vi "CRYO_MASTER_FULL_IP.vi"() -> ()   [LabVIEW 2017]
uses:
  LSI218Data.lvclass
  LSI336Data.lvclass
  USBData.lvclass
  6240AData.lvclass
  DMMsData.lvclass
  <vilib>/DAQmx/miscellaneous.llb/DAQmx Fill In Error Info.vi
  <vilib>/DAQmx/create/channels.llb/DAQmx Create Channel (DO-Digital Output).vi
  <vilib>/DAQmx/create/channels.llb/DAQmx Create Channel (AO-Voltage-Basic).vi
  <vilib>/express/express arith-compare/Formula/XNode/ExpressFormulaBlockNode.xnode
  <vilib>/Analysis/NI_AALBase.lvlib
panel:
  out "Graph 12":T1(graph) caption="XY Graph"
  out "Graph 11":T1(graph) caption="XY Graph"
  out "Graph 10":T1(graph) caption="XY Graph"
  in  "Automatic \nScreenshots?":bool=TRUE
  in  "Frontpanel screenshots":bool
  in  "Screenshots interval":i64=3605
  in  "Record interval":i64=10
  out "Cycle #":u32=4959
  in  "Measurement Interval (s)":dbl=1.0
  in  "Stop Button":bool
  in  "?":T2(tab)=enum."DIAGRAM"
  out "RUN Identifier":string="20201002_111738_PreCooling"
  in  "Base Path (screenshots)":path=path "C:/LabVIEW/DATA/Google/TUCAN Experiments/KEK_cryotests_2019-2020/data/screenshots"
  out "error out (USB6210/6218 AOUT)":errorcluster
  in  "AOUT 1 Label":string="KIKUSUI_I"
  in  "AOUT 0 Label":string="KIKUSUI_V"
  in  "DOUT Labels":string[](array[string])=["D_V1_NO", "D_V2_NC", "D_CV1"]
  in  "AOUT for Current CTRL":tag="Dev1/ao1"
  in  "AOUT For Voltage CTRL":tag="Dev1/ao0"
  out "AO task out":refnum<k21>="20201002_111738_PreCooling_AO"
  in  "Analog Out ON?":bool=TRUE
  in  "InstName (USB6218)":string="USB6218"
  in  "USB6218 Config":T3(array[cluster])=[{"Label"="F_1", "FileFormat"="%5.5f", "Active?"=TRUE, "Physical CH"="Dev1/ai0", " terminal\n type"=10083, "ConversionType"={"Type"=enum."SimpleProp", "ConversionParameters"=[0.0, 5.0, 0.0, 500.0]}, "VoltageLimits"=[0.0, 5.0]}, {"Label"="F_2", "FileFormat"="%5.5f", "Active?"=TRUE, "Physical CH"="Dev1/ai1", " terminal\n type"=10083, "ConversionType"={"Type"=enum."SimpleProp", "ConversionParameters"=[0.0, 5.0, 0.0, 200.0]}, "VoltageLimits"=[0.0, 5.0]}, {"Label"="F_3", "FileFormat"="%5.5f", "Active?"=TRUE, "Physical CH"="Dev1/ai2", " terminal\n type"=10083, "ConversionType"={"Type"=enum."SimpleProp", "ConversionParameters"=[0.0, 5.0, 0.0, 200.0]}, "VoltageLimits"=[0.0, 5.0]}, {"Label"="F_4", "FileFormat"="%5.5f", "Active?"=TRUE, "Physical CH"="Dev1/ai3", " terminal\n type"=10083, "ConversionType"={"Type"=enum."SimpleProp", "ConversionParameters"=[0.0, 5.0, 0.0, 500.0]}, "VoltageLimits"=[0.0, 5.0]}, {"Label"="F_5", "FileFormat"="%5.5f", "Active?"=TRUE, "Physical CH"="Dev1/ai4", " terminal\n type"=10083, "ConversionType"={"Type"=enum."SimpleProp", "ConversionParameters"=[0.0, 5.0, 0.0, 500.0]}, "VoltageLimits"=[0.0, 5.0]}, {"Label"="I_CV", "FileFormat"="%3.5f", "Active?"=TRUE, "Physical CH"="Dev1/ai5", " terminal\n type"=10083, "ConversionType"={"Type"=enum."Raw", "ConversionParameters"=[0.0, 0.0, 0.0, 0.0]}, "VoltageLimits"=[0.0, 10.0]}, {"Label"="CV1_answer", "FileFormat"="%3.5f", "Active?"=TRUE, "Physical CH"="Dev1/ai6", " terminal\n type"=10083, "ConversionType"={"Type"=enum."SimpleProp", "ConversionParameters"=[1.0, 5.0, 0.0, 100.0]}, "VoltageLimits"=[0.0, 5.0]}] {"terminal\n type" items=["Default"=-1, "RSE"=10083, "NRSE"=10078, "Differential"=10106, "Pseudodifferential"=12529]}
  out "error out (USB6218)":errorcluster
  out "error out (USB6210/6218 DOUT)":errorcluster
  out "DOUT task out":refnum<k21>="20201002_111738_DO"
  in  "DOUT Physical CH":tag[](array[tag])=["Dev1/port1/line0", "Dev1/port1/line1", "Dev1/port1/line2"]
  in  "Digital Out ON?":bool=TRUE
  in  "USB6210 Config":T3(array[cluster])=[{"Label"="P_ins", "FileFormat"="%5.5e", "Active?"=TRUE, "Physical CH"="Dev2/ai0", " terminal\n type"=10083, "ConversionType"={"Type"=enum."CC-10_LOG", "ConversionParameters"=[0.5, 9.0, 0.0, 1.0]}, "VoltageLimits"=[0.0, 10.0]}, {"Label"="P_4Kres", "FileFormat"="%5.5e", "Active?"=TRUE, "Physical CH"="Dev2/ai1", " terminal\n type"=10083, "ConversionType"={"Type"=enum."SimpleProp", "ConversionParameters"=[1.0, 5.0, 0.0, 200000.0]}, "VoltageLimits"=[0.0, 5.0]}, {"Label"="P_3HeIN", "FileFormat"="%5.5e", "Active?"=TRUE, "Physical CH"="Dev2/ai2", " terminal\n type"=10083, "ConversionType"={"Type"=enum."SimpleProp", "ConversionParameters"=[1.0, 5.0, 0.0, 200000.0]}, "VoltageLimits"=[0.0, 5.0]}, {"Label"="P_SldRTN", "FileFormat"="%5.5e", "Active?"=TRUE, "Physical CH"="Dev2/ai3", " terminal\n type"=10083, "ConversionType"={"Type"=enum."SimpleProp", "ConversionParameters"=[1.0, 5.0, 0.0, 200000.0]}, "VoltageLimits"=[0.0, 5.0]}, {"Label"="P_3Hepot", "FileFormat"="%5.5e", "Active?"=TRUE, "Physical CH"="Dev2/ai4", " terminal\n type"=10083, "ConversionType"={"Type"=enum."SimpleProp", "ConversionParameters"=[0.0, 10.0, 0.0, 133320.0]}, "VoltageLimits"=[0.0, 10.0]}, {"Label"="P_1Kpot", "FileFormat"="%5.5e", "Active?"=TRUE, "Physical CH"="Dev2/ai5", " terminal\n type"=10083, "ConversionType"={"Type"=enum."SimpleProp", "ConversionParameters"=[0.0, 10.0, 0.0, 133320.0]}, "VoltageLimits"=[0.0, 10.0]}, {"Label"="P_Dewar", "FileFormat"="%5.5e", "Active?"=TRUE, "Physical CH"="Dev2/ai6", " terminal\n type"=10083, "ConversionType"={"Type"=enum."SimpleProp", "ConversionParameters"=[1.0, 5.0, 0.0, 200000.0]}, "VoltageLimits"=[0.0, 5.0]}, {"Label"="DP_HEX4", "FileFormat"="%5.5e", "Active?"=TRUE, "Physical CH"="Dev2/ai7", " terminal\n type"=10083, "ConversionType"={"Type"=enum."SimpleProp", "ConversionParameters"=[1.0, 5.0, 0.0, 1000.0]}, "VoltageLimits"=[0.0, 5.0]}, {"Label"="DP_HEX5", "FileFormat"="%5.5e", "Active?"=TRUE, "Physical CH"="Dev2/ai8", " terminal\n type"=10083, "ConversionType"={"Type"=enum."SimpleProp", "ConversionParameters"=[1.0, 5.0, 0.0, 20000.0]}, "VoltageLimits"=[0.0, 5.0]}, {"Label"="L1", "FileFormat"="%5.5f", "Active?"=TRUE, "Physical CH"="Dev2/ai9", " terminal\n type"=10083, "ConversionType"={"Type"=enum."SimpleProp", "ConversionParameters"=[0.0, 10.0, 0.0, 100.0]}, "VoltageLimits"=[0.0, 10.0]}, {"Label"="L2-1", "FileFormat"="%5.5f", "Active?"=TRUE, "Physical CH"="Dev2/ai10", " terminal\n type"=10083, "ConversionType"={"Type"=enum."SimpleProp", "ConversionParameters"=[0.0, 10.0, 0.0, 100.0]}, "VoltageLimits"=[0.0, 10.0]}, {"Label"="L2-2", "FileFormat"="%5.5f", "Active?"=TRUE, "Physical CH"="Dev2/ai11", " terminal\n type"=10083, "ConversionType"={"Type"=enum."SimpleProp", "ConversionParameters"=[0.0, 10.0, 0.0, 100.0]}, "VoltageLimits"=[0.0, 10.0]}, {"Label"="L3", "FileFormat"="%5.5f", "Active?"=TRUE, "Physical CH"="Dev2/ai12", " terminal\n type"=10083, "ConversionType"={"Type"=enum."SimpleProp", "ConversionParameters"=[0.0, 10.0, 0.0, 100.0]}, "VoltageLimits"=[0.0, 10.0]}, {"Label"="P_HEX7OUT", "FileFormat"="%5.5e", "Active?"=TRUE, "Physical CH"="Dev2/ai13", " terminal\n type"=10083, "ConversionType"={"Type"=enum."SimpleProp", "ConversionParameters"=[1.0, 5.0, 0.0, 200000.0]}, "VoltageLimits"=[0.0, 5.0]}, {"Label"="P_IPHe", "FileFormat"="%5.5e", "Active?"=TRUE, "Physical CH"="Dev2/ai14", " terminal\n type"=10083, "ConversionType"={"Type"=enum."CC-10_LOG", "ConversionParameters"=[0.5, 9.0, 0.0, 1.0]}, "VoltageLimits"=[0.0, 10.0]}] {"terminal\n type" items=["Default"=-1, "RSE"=10083, "NRSE"=10078, "Differential"=10106, "Pseudodifferential"=12529]}
  in  "RUN label":string="PreCooling"
  in  "Base Path":path=path "C:/LabVIEW/DATA/Precooling/ScreenShot"
  in  "InstName (USB6210)":string="USB6210"
  out "error out (USB6210)":errorcluster
  out "File Refn USB AO":refnum<file>
  out "File Refn USB DO":refnum<file>
  out "error out (LSI336)":errorcluster
  in  "InstName (LSI336)":string="LSI336"
  in  "FileFormat (336)":string="%4.4f"
  in  "LSI336Settings(X,Y)":T4(array[cluster])=[{"LSIName"="LSi336X", "Labels"=["T1K3-1", "T1K3-2", "T3He5", "T3He8"], "SensorLocations"=[enum."T1K3-1", enum."T1K3-2", enum."T3He5", enum."T3He8"], "Active?"=TRUE, "VISA res. name"="GPIB0::6::INSTR"}, {"LSIName"="LSi336Y", "Labels"=["T3He6-1", "T3He6-2", "T3He7-1", "T3He7-2"], "SensorLocations"=[enum."T3He6-1", enum."T3He6-2", enum."T3He7-1", enum."T3He7-2"], "Active?"=TRUE, "VISA res. name"="GPIB0::2::INSTR"}]
  in  "FileFormat (218)":string="%4.4f"
  in  "InstName (LSI218)":string="LSI218"
  in  "LSI218Settings(A-F)":T4(array[cluster])=[{"LSIName"="LSI218A", "Labels"=["T3He10", "T3He1-1", "TTH3", "TTH4", "TTH1", "TTH2", "T4He1", "T1K1"], "SensorLocations"=[enum."T3He10", enum."T3He1-1", enum."TTH3", enum."TTH4", enum."TTH1", enum."TTH2", enum."T4He1", enum."T1K1"], "Active?"=TRUE, "VISA res. name"="GPIB0::7::INSTR"}, {"LSIName"="LSI218B", "Labels"=["N.C.", "N.C.", "N.C.", "N.C.", "T3He2-1", "T3He2-2", "T3He3", "T3He1-4"], "SensorLocations"=[enum."N.C.", enum."N.C.", enum."N.C.", enum."N.C.", enum."T3He2-1", enum."T3He2-2", enum."T3He3", enum."T3He1-4"], "Active?"=TRUE, "VISA res. name"="GPIB0::4::INSTR"}, {"LSIName"="LSI218C", "Labels"=["T4He3-1", "T4He3-2", "T4He3-3", "T4He3-4", "T4He2-1", "T4He2-2", "T4He4", "T4He5"], "SensorLocations"=[enum."T4He3-1", enum."T4He3-2", enum."T4He3-3", enum."T4He3-4", enum."T4He2-1", enum."T4He2-2", enum."T4He4", enum."T4He5"], "Active?"=TRUE, "VISA res. name"="GPIB0::3::INSTR"}, {"LSIName"="LSI218D", "Labels"=["T4He6", "T4He9", "T3He1-2", "T3He1-3", "T4He7", "T4He8", "T4He10", "T1K6"], "SensorLocations"=[enum."T4He6", enum."T4He9", enum."T3He1-2", enum."T3He1-3", enum."T4He7", enum."T4He8", enum."T4He10", enum."T1K6"], "Active?"=TRUE, "VISA res. name"="GPIB0::5::INSTR"}, {"LSIName"="LSI218E", "Labels"=["TIP1", "N.C.", "TIP2", "N.C.", "TIP3", "TIP4", "TIP5", "N.C."], "SensorLocations"=[enum."TIP1", enum."N.C.", enum."TIP2", enum."N.C.", enum."TIP3", enum."TIP4", enum."TIP5", enum."N.C."], "Active?"=TRUE, "VISA res. name"="GPIB0::11::INSTR"}, {"LSIName"="LSI218F", "Labels"=["T1K2", "T1K4", "T1K5", "T3He4", "T3He9", "TIP6", "N.C.", "N.C."], "SensorLocations"=[enum."T1K2", enum."T1K4", enum."T1K5", enum."T3He4", enum."T3He9", enum."TIP6", enum."N.C.", enum."N.C."], "Active?"=TRUE, "VISA res. name"="GPIB0::8::INSTR"}]
  out "error out (LSI218)":errorcluster
  out "RUN Identifier 2":string="20201002_111738_PreCooling" caption="RUN Identifier"
  out "Graph 3":T1(graph) caption="XY Graph"
  out "Graph 1":T1(graph) caption="XY Graph"
  in  "FIle suffix 4":string="Graph4_1KPot_oscillation"
  in  "Take Screenshot! 4":bool
  in  "Take Screenshot! 3":bool
  in  "Take Screenshot! 2":bool
  in  "Take Screenshot! 1":bool
  in  "FIle suffix 3":string="Graph3_1KPot_oscillation"
  in  "FIle suffix 2":string="Graph2_1KPot_oscillation"
  in  "FIle suffix 1":string="Graph1_1KPot_oscillation"
  in  "log/linear 2":bool
  in  "Tab Control 2":T5(tab)
  in  "Plot selecter (USB6210)\n    1      2     3     4":bool[][](array[boolean])=[[TRUE, FALSE, FALSE, FALSE], [TRUE, FALSE, FALSE, FALSE], [TRUE, FALSE, FALSE, FALSE], [TRUE, FALSE, FALSE, FALSE], [TRUE, FALSE, FALSE, FALSE], [TRUE, FALSE, FALSE, FALSE], [TRUE, FALSE, FALSE, FALSE], [FALSE, TRUE, FALSE, FALSE], [FALSE, TRUE, FALSE, FALSE], [FALSE, TRUE, FALSE, FALSE], [FALSE, TRUE, FALSE, FALSE], [FALSE, TRUE, FALSE, FALSE], [FALSE, TRUE, FALSE, FALSE], [TRUE, FALSE, FALSE, FALSE], [FALSE, FALSE, FALSE, FALSE], [FALSE, FALSE, FALSE, FALSE]]
  out "All Labels (USB6210)":string[](array[string])=["P_ins", "P_4Kres", "P_3HeIN", "P_SldRTN", "P_3Hepot", "P_1Kpot", "P_Dewar", "DP_HEX4", "DP_HEX5", "L1", "L2-1", "L2-2", "L3", "P_HEX7OUT"]
  out "Last Data \n(USB6210)":dbl[](array[numeric])=[0.00015623126743967978, 102646.15993978488, 3637.6504873774197, 101891.36809168091, 4295.356268996977, 845.3614360135382, 101097.11052150725, -5.334954304017453, 66.29225516513348, 99.98613335417497, 67.02762914376657, 60.52032349741818, 48.99728244152156, 103856.45826569716] format="%#_6e"
  out "Time of Last Measurement (USB6210)":timestamp=timestamp(3684454864.3849993 s since 1904-01-01)
  out "USB6210 Status":T6(ring)=enum."Ready"
  out "Last Vol\n(USB6210)":dbl[](array[numeric])=[5.596883978015126, 3.0529231987956975, 1.0727530097475484, 3.0378273618336182, 0.32218393856863015, 0.06340844854586995, 3.021942210430145, 0.9786601827839302, 1.0132584510330267, 9.998613335417497, 6.702762914376658, 6.052032349741818, 4.899728244152156, 3.077129165313943] format="%_5f"
  out "Time of Last Measurement (USB6218)":timestamp=timestamp(3684454864.391945 s since 1904-01-01)
  out "USB6218 Status":T6(ring)=enum."Ready"
  out "Last Vol \n(USB6218)":dbl[](array[numeric])=[0.4328486013755781, 0.2856827409675284, 0.008941174623972741, -0.06513496143958923, 0.9306675842076008, -6.309670101250775e-05, -0.00046218726464117564] format="%_5f"
  out "Last Data \n(USB6218)":dbl[](array[numeric])=[43.284860137557814, 11.427309638701136, 0.3576469849589097, -6.513496143958923, 93.06675842076008, -6.309670101250775e-05, -25.011554681616026] format="%#_6e"
  out "All Labels (USB6218)":string[](array[string])=["F_1", "F_2", "F_3", "F_4", "F_5", "I_CV", "CV1_answer"]
  in  "Plot selecter (USB6218)\n    1      2     3     4":bool[][](array[boolean])=[[FALSE, FALSE, TRUE, FALSE], [FALSE, FALSE, TRUE, FALSE], [FALSE, FALSE, TRUE, FALSE], [FALSE, FALSE, TRUE, FALSE], [FALSE, FALSE, TRUE, FALSE], [FALSE, FALSE, TRUE, FALSE], [FALSE, FALSE, FALSE, FALSE], [FALSE, FALSE, TRUE, FALSE], [FALSE, FALSE, TRUE, FALSE], [FALSE, FALSE, FALSE, TRUE], [FALSE, FALSE, FALSE, TRUE], [FALSE, FALSE, FALSE, TRUE], [FALSE, FALSE, FALSE, TRUE], [FALSE, FALSE, FALSE, FALSE], [FALSE, FALSE, FALSE, FALSE], [FALSE, FALSE, FALSE, FALSE]]
  out "Time of Last Measurement (LSI218)":timestamp=timestamp(3684454864.3849993 s since 1904-01-01)
  out "LSI218 Status":T7(ring)=enum."Measuring"
  out "Last Data \nLSI218 (1)":dbl[](array[numeric])=[174.86, 119.03, 131.93, 123.27, 24.68, 25.174, 4.416, 4.607, 30.0, 0.0, 0.0, 0.0, 66.96, 49.172, 4.786, 225.14, 190.27, 196.43, 244.83, 249.59, 17.993, 18.993, 22.964, 24.809]
  out "Labels LSI218 (1)":string[](array[string])=["T3He10", "T3He1-1", "TTH3", "TTH4", "TTH1", "TTH2", "T4He1", "T1K1", "N.C.", "N.C.", "N.C.", "N.C.", "T3He2-1", "T3He2-2", "T3He3", "T3He1-4", "T4He3-1", "T4He3-2", "T4He3-3", "T4He3-4", "T4He2-1", "T4He2-2", "T4He4", "T4He5"]
  in  "Plot selecter LSI218(1)\n    1      2     3     4":bool[][](array[boolean])=[[FALSE, FALSE, FALSE, FALSE], [FALSE, FALSE, FALSE, FALSE], [FALSE, FALSE, FALSE, TRUE], [FALSE, FALSE, FALSE, TRUE], [FALSE, FALSE, FALSE, TRUE], [FALSE, FALSE, FALSE, TRUE], [FALSE, FALSE, FALSE, TRUE], [FALSE, FALSE, FALSE, TRUE], [FALSE, FALSE, FALSE, FALSE], [FALSE, FALSE, FALSE, FALSE], [FALSE, FALSE, FALSE, FALSE], [FALSE, FALSE, FALSE, FALSE], [FALSE, FALSE, FALSE, TRUE], [FALSE, FALSE, FALSE, TRUE], [FALSE, FALSE, FALSE, FALSE], [FALSE, FALSE, FALSE, FALSE], [FALSE, FALSE, FALSE, TRUE], [FALSE, FALSE, FALSE, TRUE], [FALSE, FALSE, FALSE, TRUE], [FALSE, FALSE, FALSE, TRUE], [FALSE, FALSE, FALSE, TRUE], [FALSE, FALSE, FALSE, TRUE], [FALSE, FALSE, FALSE, TRUE], [FALSE, FALSE, FALSE, FALSE]]
  out "Active?\n (1)":bool[](array[boolean])=[TRUE, TRUE, TRUE, TRUE, TRUE, TRUE, TRUE, TRUE, TRUE, TRUE, TRUE, TRUE, TRUE, TRUE, TRUE, TRUE, TRUE, TRUE, TRUE, TRUE, TRUE, TRUE, TRUE, TRUE]
  out "Labels LSI218 (2)":string[](array[string])=["T4He6", "T4He9", "T3He1-2", "T3He1-3", "T4He7", "T4He8", "T4He10", "T1K6", "TIP1", "N.C.", "TIP2", "N.C.", "TIP3", "TIP4", "TIP5", "N.C.", "T1K2", "T1K4", "T1K5", "T3He4", "T3He9", "TIP6", "N.C.", "N.C."]
  out "Active?\n(2)":bool[](array[boolean])=[TRUE, TRUE, TRUE, TRUE, TRUE, TRUE, TRUE, TRUE, TRUE, TRUE, TRUE, TRUE, TRUE, TRUE, TRUE, TRUE, TRUE, TRUE, TRUE, TRUE, TRUE, TRUE, TRUE, TRUE]
  out "Last Data \nLSI218 (2)":dbl[](array[numeric])=[26.249, 111.49, 133.91, 219.75, 133.21, 138.02, 218.7, 58.064, 250.36, 0.0, 110.28, 688.49, 56.993, 6.89, 10.053, 688.58, 1.955, 1.89, 4.175, 2.013, 2.158, 18.589, 0.433, 0.0]
  in  "Plot selecter LSI218(2)\n    1      2     3     4":bool[][](array[boolean])=[[FALSE, FALSE, FALSE, FALSE], [FALSE, FALSE, FALSE, FALSE], [FALSE, FALSE, FALSE, FALSE], [FALSE, FALSE, FALSE, FALSE], [FALSE, FALSE, FALSE, FALSE], [FALSE, FALSE, FALSE, FALSE], [FALSE, FALSE, FALSE, FALSE], [FALSE, FALSE, FALSE, FALSE], [FALSE, FALSE, FALSE, FALSE], [FALSE, FALSE, FALSE, FALSE], [FALSE, FALSE, FALSE, FALSE], [FALSE, FALSE, FALSE, FALSE], [FALSE, FALSE, FALSE, FALSE], [FALSE, FALSE, FALSE, FALSE], [FALSE, FALSE, FALSE, FALSE], [FALSE, FALSE, FALSE, FALSE], [FALSE, FALSE, FALSE, TRUE], [FALSE, FALSE, FALSE, TRUE], [FALSE, FALSE, FALSE, TRUE], [FALSE, FALSE, FALSE, FALSE], [FALSE, FALSE, FALSE, FALSE], [FALSE, FALSE, FALSE, FALSE], [FALSE, FALSE, FALSE, FALSE], [FALSE, FALSE, FALSE, FALSE]]
  in  "Plot selecter LSI336 \n     1      2     3     4":bool[][](array[boolean])=[[FALSE, FALSE, FALSE, TRUE], [FALSE, FALSE, FALSE, TRUE], [FALSE, FALSE, FALSE, TRUE], [FALSE, FALSE, FALSE, TRUE], [FALSE, FALSE, FALSE, TRUE], [FALSE, FALSE, FALSE, TRUE], [FALSE, FALSE, FALSE, TRUE], [FALSE, FALSE, FALSE, TRUE]]
  out "Time of Last Measurement (LSI336)":timestamp=timestamp(3684454864.3849993 s since 1904-01-01)
  out "Last Data \nLSI336":dbl[](array[numeric])=[1.5337, 1.5296, 1.8153, 2.1079, 2.1163, 2.122, 2.1204, 2.1198]
  out "Active?\n(LSI336)":bool[](array[boolean])=[TRUE, TRUE, TRUE, TRUE, TRUE, TRUE, TRUE, TRUE]
  out "Labels LSI336":string[](array[string])=["T1K3-1", "T1K3-2", "T3He5", "T3He8", "T3He6-1", "T3He6-2", "T3He7-1", "T3He7-2"]
  out "LSI336 Status":T7(ring)=enum."Measuring"
  in  "log/linear 1":bool=TRUE
  out "Graph 2":T1(graph) caption="XY Graph"
  out "Graph 4":T1(graph) caption="XY Graph"
  in  "log/linear 4":bool
  in  "log/linear 3":bool
  out "RUN Identifier 3":string="20201002_111738_PreCooling" caption="RUN Identifier"
  out "RUN Identifier 4":string="20201002_111738_PreCooling" caption="RUN Identifier"
  out "Fill (false)":bool=TRUE
  in  "Fill state":bool
  out "state 1 (false)":bool=TRUE
  out "state 1":bool
  out "state 2":bool
  out "state 2 (false)":bool=TRUE
  out "Status V2 CTRL":enum16{"Pressurize", "Release"}(ring)
  out "Status V1 CTRL":enum16{"Pressurize", "Release"}(ring)
  out "Lav (%)":dbl=71.20324134668614 format="%0.2f"
  out "Lstd":dbl=0.006921328322954857 format="%0.2f"
  out "Last N M.A. Levels":dbl[](array[numeric])=[71.21069849829522, 71.21168495646573, 71.21563078793135, 71.20971204069737, 71.19803895584928, 71.19672367846871, 71.19162697956635, 71.19771013641974, 71.20247801612076, 71.19951864246737, 71.19738131717675, 71.2023136066108, 71.20675266705979, 71.20510857047677] format="%_5e"
  out "Lstd history":dbl(graph)=0.007035562623226079
  out "Lav history":dbl(graph)=71.20346447405132
  out "Target Index (L)":i32=12
  in  "Auto Fll\nHe level label":string="L3"
  out "Target Index (P)":i32=6
  in  "Auto Fll\nDewar P. label":string="P_Dewar"
  out "He Level":T8(graph)=[{"TimeArray"=[timestamp(3684373440.273899 s since 1904-01-01), timestamp(3684373441.2730346 s since 1904-01-01), timestamp(3684373442.273437 s since 1904-01-01), timestamp(3684373443.273284 s since 1904-01-01), timestamp(3684373444.272991 s since 1904-01-01), timestamp(3684373445.2752414 s since 1904-01-01), timestamp(3684373446.273977 s since 1904-01-01), timestamp(3684373447.275109 s since 1904-01-01), timestamp(3684373448.275254 s since 1904-01-01), timestamp(3684373449.2756577 s since 1904-01-01), timestamp(3684373450.4052033 s since 1904-01-01), timestamp(3684373451.404408 s since 1904-01-01), timestamp(3684373452.4054728 s since 1904-01-01), timestamp(3684373453.4055552 s since 1904-01-01)], "Filtered X"=[71.22204276382959, 71.21217818635228, 71.21283582343595, 71.19179138917168, 71.17535042443726, 71.20691707682998, 71.19244902782646, 71.21612401658533, 71.1944219432413, 71.1950795822164, 71.18389972666398, 71.2358531743215, 71.21217818503723, 71.18850319588435]}, {"TimeArray"=[timestamp(3684373440.273899 s since 1904-01-01), timestamp(3684373441.2730346 s since 1904-01-01), timestamp(3684373442.273437 s since 1904-01-01), timestamp(3684373443.273284 s since 1904-01-01), timestamp(3684373444.272991 s since 1904-01-01), timestamp(3684373445.2752414 s since 1904-01-01), timestamp(3684373446.273977 s since 1904-01-01), timestamp(3684373447.275109 s since 1904-01-01), timestamp(3684373448.275254 s since 1904-01-01), timestamp(3684373449.2756577 s since 1904-01-01), timestamp(3684373450.4052033 s since 1904-01-01), timestamp(3684373451.404408 s since 1904-01-01), timestamp(3684373452.4054728 s since 1904-01-01), timestamp(3684373453.4055552 s since 1904-01-01)], "Filtered X"=[71.21069849829522, 71.21168495646573, 71.21563078793135, 71.20971204069737, 71.19803895584928, 71.19672367846871, 71.19162697956635, 71.19771013641974, 71.20247801612076, 71.19951864246737, 71.19738131717675, 71.2023136066108, 71.20675266705979, 71.20510857047677]}] caption="XY Graph"
  in  "P_safelimit_high (Pa)":dbl=300000.0 format="%_4e"
  in  "P_safelimit_low (Pa)":dbl=100.0 format="%_4e"
  in  "Auto Fill ON?":bool
  out "Pstd history":dbl(graph)=271.0714505072834
  out "Pav history":dbl(graph)=125228.66056725154
  in  "Mov. Avg Interval":i64=4
  in  "V2 (N.C.)":bool
  in  "V1 (N.O.)":bool=TRUE
  in  "N for sampling":i64=7
  in  "L_low (%)":dbl=60.0 format="%_3f"
  in  "L_high (%)":dbl=80.0 format="%_3g"
  in  "P_2_low (Pa)":dbl=125000.0 format="%_4e"
  in  "P_1_low (Pa)":dbl=135000.0 format="%_4g"
  in  "P_2_high (Pa)":dbl=135000.0 format="%_4e"
  in  "P_1_high (Pa)":dbl=140000.0 format="%_4e"
  out "Dewar Pressure":T8(graph)=[{"TimeArray"=[timestamp(3684373440.273899 s since 1904-01-01), timestamp(3684373441.2730346 s since 1904-01-01), timestamp(3684373442.273437 s since 1904-01-01), timestamp(3684373443.273284 s since 1904-01-01), timestamp(3684373444.272991 s since 1904-01-01), timestamp(3684373445.2752414 s since 1904-01-01), timestamp(3684373446.273977 s since 1904-01-01), timestamp(3684373447.275109 s since 1904-01-01), timestamp(3684373448.275254 s since 1904-01-01), timestamp(3684373449.2756577 s since 1904-01-01), timestamp(3684373450.4052033 s since 1904-01-01), timestamp(3684373451.404408 s since 1904-01-01), timestamp(3684373452.4054728 s since 1904-01-01), timestamp(3684373453.4055552 s since 1904-01-01)], "Filtered X"=[126288.14675345753, 125406.72915551426, 125684.63887820412, 125234.06378922188, 125026.86502899571, 125252.15243360576, 124413.49040192305, 124206.29196931639, 125817.83836590881, 125184.73094394046, 125132.10848420773, 125707.66108196737, 125227.48582278784, 126493.70118827428]}, {"TimeArray"=[timestamp(3684373440.273899 s since 1904-01-01), timestamp(3684373441.2730346 s since 1904-01-01), timestamp(3684373442.273437 s since 1904-01-01), timestamp(3684373443.273284 s since 1904-01-01), timestamp(3684373444.272991 s since 1904-01-01), timestamp(3684373445.2752414 s since 1904-01-01), timestamp(3684373446.273977 s since 1904-01-01), timestamp(3684373447.275109 s since 1904-01-01), timestamp(3684373448.275254 s since 1904-01-01), timestamp(3684373449.2756577 s since 1904-01-01), timestamp(3684373450.4052033 s since 1904-01-01), timestamp(3684373451.404408 s since 1904-01-01), timestamp(3684373452.4054728 s since 1904-01-01), timestamp(3684373453.4055552 s since 1904-01-01)], "Filtered X"=[125428.10696888957, 125511.97316498918, 125422.7625555792, 125653.39464409945, 125338.074212984, 125299.43003250686, 124981.6429134366, 124724.69995846022, 124922.4432926885, 124905.58792027218, 125085.24244084334, 125460.58471900609, 125312.99658322585, 125640.23914430931]}] caption="XY Graph"
  out "Last N M.A. Pressures":dbl[](array[numeric])=[125428.10696888957, 125511.97316498918, 125422.7625555792, 125653.39464409945, 125338.074212984, 125299.43003250686, 124981.6429134366, 124724.69995846022, 124922.4432926885, 124905.58792027218, 125085.24244084334, 125460.58471900609, 125312.99658322585, 125640.23914430931] format="%_5e"
  out "Pav (Pa)":dbl=125263.36989652073 format="%0.4e"
  out "Pstd":dbl=291.18311466125465 format="%0.4e"
  out "File Refn DewarCTRL":refnum<file>
  out "Error Out (Dewar CTRL":errorcluster
  in  "update values":bool
  out "Monitor Current (mA)":dbl=-0.5520142344653531 min=0.0 max=1.9 format="%_4e"
  in  "update current":bool
  out "USB AOUT":dbl[](array[numeric])=[12.0, 4.0, 0.18461538461538463, 0.06969546425555169]
  out "Graph 7":T9(graph) caption="XY Graph"
  in  "upper limit (V)\n (Kikusui)":dbl=12.0 format="%_3f"
  in  "lower limit (V) \n(Kikusui)":dbl format="%_3f"
  in  "lower limit (mA) \n(Kikusui)":dbl=4.0 format="%_3f"
  in  "upper limit (mA)\n (Kikusui)":dbl=40.0 format="%_3f"
  in  "lower limit (mA)":dbl=4.0 format="%_3f"
  in  "SetCurrent 2 (mA)":dbl=4.0 min=4.0 max=500.0 format="%_3f"
  in  "upper limit (mA)":dbl=500.0 format="%_3f"
  out "error out (KIKUSI CTRL)":errorcluster
  out "ActualVoltage (V)":dbl[](array[numeric]) format="%_6g"
  out "ActualCurrent (A)":dbl[](array[numeric])=[0.01, 0.0] format="%_3e"
  in  "SetCurrent 1 (mA)":dbl=4.0 min=4.0 max=500.0 format="%_3g"
  in  "Output\n (ADCMT)":bool[](array[boolean])=[FALSE, FALSE]
  out "error out (ADCMT6420A)":errorcluster
  in  "Voltage limits (V)":dbl[](array[numeric])=[12.0, 12.0] format="%_3f"
  in  "CtrlLabels":string[](array[string])=["CV2", "CV3"]
  in  "VISA":refnum<visa-resource-name>[](array[refnum])=["GPIB0::1::INSTR", "GPIB0::12::INSTR"]
  out "Initialized?":bool
  in  "InstName":string="ADCMT6240"
  out "Graph 6":T8(graph)=[{"TimeArray"=[timestamp(3684448950.65012 s since 1904-01-01), timestamp(3684448954.168732 s since 1904-01-01), timestamp(3684448960.15376 s since 1904-01-01)], "Filtered X"=[0.8, 0.8, 0.01]}, {"TimeArray"=[timestamp(3684448950.65012 s since 1904-01-01), timestamp(3684448954.168732 s since 1904-01-01), timestamp(3684448960.15376 s since 1904-01-01)], "Filtered X"=[0.0, 0.0, 0.0]}, {"TimeArray"=[timestamp(3684448950.65012 s since 1904-01-01), timestamp(3684448954.168732 s since 1904-01-01), timestamp(3684448960.15376 s since 1904-01-01)], "Filtered X"=[0.8, 0.8, 0.01]}, {"TimeArray"=[timestamp(3684448950.65012 s since 1904-01-01), timestamp(3684448954.168732 s since 1904-01-01), timestamp(3684448960.15376 s since 1904-01-01)], "Filtered X"=[0.0, 0.0, 0.0]}] caption="XY Graph"
  in  "Initialize":bool
  in  "CONTROL KIKUSUI?":bool=TRUE
  in  "OUTPUT\n(Kikusui)":bool
  in  "Set Voltage (V)\n (Kikusui)":dbl=12.0 min=0.0 max=12.0 format="%_3g"
  in  "Set Current (mA)\n (Kikusui)":dbl=4.0 min=4.0 max=40.0 format="%_3g"
  out "RUN Identifier 5":string="20201002_111738_PreCooling" caption="RUN Identifier"
  in  "Measure DMMs?":bool
  out "DMMsLabels":string[](array[string])=["V_H2", "V_H4", "I_H2", "I_H4"]
  out "Active?":bool[](array[boolean])=[TRUE, FALSE, TRUE, FALSE]
  out "DMM LastMeasurements":dbl[](array[numeric])=[2.6334599999999997e-05, 0.0, 0.0, 0.0]
  out "Graph DMMs 2":T1(graph) caption="XY Graph"
  out "DMMFileName":string="20201001_162428_PreCooling_DMMs_20201001_162516.csv"
  out "error out (DMMs)":errorcluster
  out "cycle # (DMMs)":i32=10009
  in  "DMMsConfig":T10(array[cluster])=[{"Label"="V_H2", "Active?"=TRUE, "VISA resource name"="GPIB0::22::INSTR", "Device"=enum."Agilent34401A", "Measurement"=enum."DC Volts", "FileFormat"="%4.6e"}, {"Label"="V_H4", "Active?"=FALSE, "VISA resource name"="USB0::0x1334::0x0204::262800451::INSTR", "Device"=enum."ADCMT7351", "Measurement"=enum."DC Volts", "FileFormat"="%4.6e"}, {"Label"="I_H2", "Active?"=TRUE, "VISA resource name"="USB0::0x1334::0x0204::262800066::INSTR", "Device"=enum."ADCMT7351", "Measurement"=enum."DC Currents", "FileFormat"="%4.4e"}, {"Label"="I_H4", "Active?"=FALSE, "VISA resource name"="GPIB0::23::INSTR", "Device"=enum."HP3478A", "Measurement"=enum."DC Currents", "FileFormat"="%4.4e"}]
  in  "Measurement Interval DMMs (ms)":i64=500
  in  "InstName DMMs":string="DMMs"
  in  "Initialize (DMMs)":bool
  out "Graph DMMs 1":T1(graph) caption="XY Graph"
  out "error out (DMM graphs)":errorcluster
  in  "Sample #":i32=5
  in  "IPHe pressure":string="P_IPHe"
  out "P (IPHe)":dbl=102813.89149070326 format="%_4e"
  out "P_IPHe":dbl=102813.89149070326 format="%_4e"
  out "P_HEX7OUT":dbl=102813.89149070326 format="%_4e"
  out "P (HEX7 out)":dbl=102813.89149070326 format="%_4e"
  out "DP HEX5":dbl=83.0651823977413 format="%_4e"
  out "DP_HEX5":dbl=83.0651823977413 format="%_4e"
  in  "Diff pressure HEX5":string="DP_HEX5"
  out "3He pot level":dbl=100.01835834612064 format="%_4f"
  in  "3He pot":string="L1"
  out "He level (3He)":dbl(slide)=100.01835834612064 scale=0.0..100.0
  out "He level (1K) b":dbl(slide)=60.44995659847142 scale=0.0..100.0
  out "He level (1K)":dbl(slide)=66.98422510636897 scale=0.0..100.0
  out "He level (4K)":dbl(slide)=48.990048499529806 scale=0.0..100.0
  out "1K pot(b1)":dbl=60.44995659847142 format="%_4f"
  in  "1K pot (b)":string="L2-2"
  in  "1K pot level":string="L2-1"
  out "L(1K) (a1)":dbl=66.98422510636897 format="%_4f"
  in  "SensorLocation 2":T11(ring)=enum."T3He5"
  out "Temperature 2":dbl=1.7995
  out "DP HEX4":dbl=-5.3760643808830615 format="%_4e"
  in  "Diff pressure HEX4":string="DP_HEX4"
  out "V2":bool
  out "V1":bool=TRUE
  out "F5 (3He pump ex.)":dbl=93.69145685771404 format="%_4f"
  out "F4 (3He in to HEX7)":dbl=-6.1879951345084425 format="%_3f"
  out "F3 (4He rtn flw via HEX7)":dbl=0.443132092574638 format="%_4f"
  out "F1 (1K pump exhaust) flow":dbl=43.19279928269202 format="%_4f"
  out "P (Dewar)":dbl=101207.2871705193 format="%_4e"
  out "P (1K pot)":dbl=854.1288946139209 format="%_4e"
  out "P (3He pot)":dbl=4268.177149245784 format="%_4e"
  out "P (shield return)":dbl=102073.89943522238 format="%_4e"
  out "P (3He IN)":dbl=3879.377992445654 format="%_4e"
  out "P (4K reservoir)":dbl=102544.20548859666 format="%_4e"
  out "P (insulation)":dbl=0.00015646802075869302 format="%_4e"
  in  "3He pump exhaust flow":string="F_5"
  out "F_5":dbl=93.69145685771404 format="%_4f"
  in  "3He incoming flow into HEX7":string="F_4"
  out "F_4":dbl=-6.1879951345084425 format="%_4f"
  out "F_3":dbl=0.443132092574638 format="%_4f"
  in  "4He return flow from HEX7":string="F_3"
  out "F_2":dbl=11.32341237657438 format="%_4f"
  in  "Shield flow":string="F_2"
  out "P_SldRTN":dbl=102073.89943522238 format="%_4e"
  in  "3He pot pressure":string="P_3Hepot"
  out "P_3Hepot":dbl=4268.177149245784 format="%_4e"
  in  "Shield return press.":string="P_SldRTN"
  out "F_1":dbl=43.19279928269202 format="%_4f"
  in  "1K pump exhaust flow":string="F_1"
  out "P_Dewar":dbl=101207.2871705193 format="%_4e"
  in  "Dewar pressure":string="P_Dewar"
  out "P_1Kpot":dbl=854.1288946139209 format="%_4e"
  in  "1Kpot pressure":string="P_1Kpot"
  out "P_3HeIN":dbl=3879.377992445654 format="%_4e"
  in  "3He inlet pressure":string="P_3HeIN"
  in  "4K reservoir pressure":string="P_4Kres"
  out "P_4Kres":dbl=102544.20548859666 format="%_4e"
  out "P_ins":dbl=0.00015646802075869302 format="%_4e"
  in  "Insulation vacuum":string="P_ins"
  out "T3He7-1/6-2 (3He pot) 2":dbl=2.1199 format="%_4f"
  out "T3He7-1/7-2 (HEX1)":dbl=2.1206 format="%_4f"
  out "T3He6-1/6-2 (3He pot) 2":dbl=2.1224 format="%_4f"
  out "T3He6-1/6-2 (HEX1)":dbl=2.1167 format="%_4f"
  out "T1K3-1/3-2 (1K pot) 2":dbl=1.53 format="%_4f"
  out "T1K3-1/3-2 (1K pot)":dbl=1.5341 format="%_4f"
  out "T4He1 (4K reservoir )":dbl=4.418 format="%_4f"
  out "Temperature 1":dbl=25.175
  in  "SensorLocation 1":T11(ring)=enum."TTH2"
  out "TIP7":dbl format="%_4g"
  out "T3He6-2":dbl=2.1224 format="%_4g"
  out "T3He7-2":dbl=2.1199 format="%_4g"
  out "T3He6-1":dbl=2.1167 format="%_4g"
  out "T3He4":dbl=2.021 format="%_4g"
  out "T3He7-1":dbl=2.1206 format="%_4g"
  out "T3He8":dbl=2.1078 format="%_4g"
  out "T3He5":dbl=1.7995 format="%_4g"
  out "T1K3-2":dbl=1.53 format="%_4g"
  out "T1K3-1":dbl=1.5341 format="%_4g"
  out "TIP6":dbl=18.591 format="%_4g"
  out "T3He9":dbl=2.146 format="%_4g"
  out "T1K5":dbl=4.181 format="%_4g"
  out "T1K4":dbl=1.897 format="%_4g"
  out "T1K2":dbl=1.952 format="%_4g"
  out "TIP5":dbl=10.064 format="%_4g"
  out "TIP4":dbl=6.894 format="%_4g"
  out "TIP3":dbl=56.992 format="%_4g"
  out "TIP2":dbl=110.28 format="%_4g"
  out "TIP1":dbl=250.37 format="%_4g"
  out "T1K6":dbl=58.037 format="%_4g"
  out "T4He10":dbl=218.68 format="%_4g"
  out "T4He8":dbl=138.02 format="%_4g"
  out "T4He7":dbl=133.22 format="%_4g"
  out "T3He1-3":dbl=219.72 format="%_4g"
  out "T3He1-2":dbl=133.83 format="%_4g"
  out "T4He9":dbl=111.48 format="%_4g"
  out "T4He6":dbl=26.241 format="%_4g"
  out "T4He5":dbl=24.814 format="%_4g"
  out "T4He4":dbl=22.962 format="%_4g"
  out "T4He2-2":dbl=19.013 format="%_4g"
  out "T4He2-1":dbl=17.972 format="%_4g"
  out "T4He3-4":dbl=249.58 format="%_4g"
  out "T4He3-3":dbl=244.82 format="%_4g"
  out "T4He3-2":dbl=196.4 format="%_4g"
  out "T4He3-1":dbl=190.21 format="%_4g"
  out "T3He1-4":dbl=225.11 format="%_4g"
  out "T3He3":dbl=4.771 format="%_4g"
  out "T3He2-2":dbl=49.183 format="%_4g"
  out "T3He2-1":dbl=66.962 format="%_4g"
  out "T1K1":dbl=4.591 format="%_4g"
  out "T4He1":dbl=4.418 format="%_4g"
  out "TTH1":dbl=24.68 format="%_4g"
  out "TTH2":dbl=25.175 format="%_4g"
  out "TTH4":dbl=123.27 format="%_4g"
  out "TTH3":dbl=131.91 format="%_4g"
  out "T3He1-1":dbl=118.93 format="%_4g"
  out "T3He10":dbl=174.85 format="%_4g"
  out "F2 (shield flow)":dbl=11.32341237657438 format="%_4f"
  out "DP_HEX4":dbl=-5.3760643808830615 format="%_4e"
  in  "4K reservoir level":string="L3"
  out "L3":dbl=48.990048499529806 format="%_4f"
  out "RUN Identifier 6":string="20201002_111738_PreCooling" caption="RUN Identifier"
  in  "HEX7 out pressure":string="P_HEX7OUT"
  out "Series 1":string[](array[string])=["P_ins", "P_4Kres", "P_3HeIN", "P_SldRTN", "P_3Hepot", "P_1Kpot", "P_Dewar", "P_HEX7OUT"]
  out "Series 2":string[](array[string])=["DP_HEX4", "DP_HEX5", "L1", "L2-1", "L2-2", "L3"]
  out "Series 3":string[](array[string])=["F_1", "F_2", "F_3", "F_4", "F_5", "I_CV"]
  out "Series 4":string[](array[string])=["TTH3", "TTH4", "TTH1", "TTH2", "T4He1", "T1K1", "T3He2-1", "T3He2-2", "T4He3-1", "T4He3-2", "T4He3-3", "T4He3-4", "T4He2-1", "T4He2-2", "T4He4", "T1K2", "T1K4", "T1K5", "T1K3-1", "T1K3-2", "T3He5", "T3He8", "T3He6-1", "T3He6-2", "T3He7-1", "T3He7-2"]
  out "Plot errors":errorcluster
  out "LastMeasurementConfig (218)":T12(array[cluster])=[{"LSIName"="LSI218A", "Active?"=TRUE, "LastData"=[174.86, 119.03, 131.93, 123.27, 24.68, 25.174, 4.416, 4.607], "Labels"=["T3He10", "T3He1-1", "TTH3", "TTH4", "TTH1", "TTH2", "T4He1", "T1K1"]}, {"LSIName"="LSI218B", "Active?"=TRUE, "LastData"=[30.0, 0.0, 0.0, 0.0, 66.96, 49.172, 4.786, 225.14], "Labels"=["N.C.", "N.C.", "N.C.", "N.C.", "T3He2-1", "T3He2-2", "T3He3", "T3He1-4"]}, {"LSIName"="LSI218C", "Active?"=TRUE, "LastData"=[190.27, 196.43, 244.83, 249.59, 17.993, 18.993, 22.964, 24.809], "Labels"=["T4He3-1", "T4He3-2", "T4He3-3", "T4He3-4", "T4He2-1", "T4He2-2", "T4He4", "T4He5"]}, {"LSIName"="LSI218D", "Active?"=TRUE, "LastData"=[26.249, 111.49, 133.91, 219.75, 133.21, 138.02, 218.7, 58.064], "Labels"=["T4He6", "T4He9", "T3He1-2", "T3He1-3", "T4He7", "T4He8", "T4He10", "T1K6"]}, {"LSIName"="LSI218E", "Active?"=TRUE, "LastData"=[250.36, 0.0, 110.28, 688.49, 56.993, 6.89, 10.053, 688.58], "Labels"=["TIP1", "N.C.", "TIP2", "N.C.", "TIP3", "TIP4", "TIP5", "N.C."]}, {"LSIName"="LSI218F", "Active?"=TRUE, "LastData"=[1.955, 1.89, 4.175, 2.013, 2.158, 18.589, 0.433, 0.0], "Labels"=["T1K2", "T1K4", "T1K5", "T3He4", "T3He9", "TIP6", "N.C.", "N.C."]}]
  out "DataArrayConv (USB6210)":dbl[][](array[numeric])
  out "LastMeasurementConfig (336)":T12(array[cluster])=[{"LSIName"="LSi336X", "Active?"=TRUE, "LastData"=[1.5337, 1.5296, 1.8153, 2.1079], "Labels"=["T1K3-1", "T1K3-2", "T3He5", "T3He8"]}, {"LSIName"="LSi336Y", "Active?"=TRUE, "LastData"=[2.1163, 2.122, 2.1204, 2.1198], "Labels"=["T3He6-1", "T3He6-2", "T3He7-1", "T3He7-2"]}]
  out "DataArrayConv (USB6218)":dbl[][](array[numeric])
  out "TimeArray (USB6218)":timestamp[](array[timestamp])
  out "Data Array sizes (6210)":i32[](array[numeric])=[4959, 14]
  out "DataArraySize (6218)":i32[](array[numeric])=[4959, 7]
  out "TimeArray size (6218)":i32=4959
  out "TimeArray (LSI336)":timestamp[](array[timestamp])
  out "TimeArray Size (336)":i32=4959
  out "DataArray (336)":dbl[][](array[numeric])
  out "DataArray size (336)":i32[](array[numeric])=[4959, 8]
  out "LastData (LSI218)":dbl[](array[numeric])=[174.86, 119.03, 131.93, 123.27, 24.68, 25.174, 4.416, 4.607, 30.0, 0.0, 0.0, 0.0, 66.96, 49.172, 4.786, 225.14, 190.27, 196.43, 244.83, 249.59, 17.993, 18.993, 22.964, 24.809, 26.249, 111.49, 133.91, 219.75, 133.21, 138.02, 218.7, 58.064, 250.36, 0.0, 110.28, 688.49, 56.993, 6.89, 10.053, 688.58, 1.955, 1.89, 4.175, 2.013, 2.158, 18.589, 0.433, 0.0]
  out "TempSensorsLocations":T13(array[ring])=[enum."T3He10", enum."T3He1-1", enum."TTH3", enum."TTH4", enum."TTH1", enum."TTH2", enum."T4He1", enum."T1K1", enum."N.C.", enum."N.C.", enum."N.C.", enum."N.C.", enum."T3He2-1", enum."T3He2-2", enum."T3He3", enum."T3He1-4", enum."T4He3-1", enum."T4He3-2", enum."T4He3-3", enum."T4He3-4", enum."T4He2-1", enum."T4He2-2", enum."T4He4", enum."T4He5", enum."T4He6", enum."T4He9", enum."T3He1-2", enum."T3He1-3", enum."T4He7", enum."T4He8", enum."T4He10", enum."T1K6", enum."TIP1", enum."N.C.", enum."TIP2", enum."N.C.", enum."TIP3", enum."TIP4", enum."TIP5", enum."N.C.", enum."T1K2", enum."T1K4", enum."T1K5", enum."T3He4", enum."T3He9", enum."TIP6", enum."N.C.", enum."N.C.", enum."T1K3-1", enum."T1K3-2", enum."T3He5", enum."T3He8", enum."T3He6-1", enum."T3He6-2", enum."T3He7-1", enum."T3He7-2"]
  out "AllTemperatures":dbl[](array[numeric])=[174.85, 118.93, 131.91, 123.27, 24.68, 25.175, 4.418, 4.591, 30.0, 0.0, 0.0, 0.0, 66.962, 49.183, 4.771, 225.11, 190.21, 196.4, 244.82, 249.58, 17.972, 19.013, 22.962, 24.814, 26.241, 111.48, 133.83, 219.72, 133.22, 138.02, 218.68, 58.037, 250.37, 0.0, 110.28, 688.49, 56.992, 6.894, 10.064, 688.58, 1.952, 1.897, 4.181, 2.021, 2.146, 18.591, 0.433, 0.0, 1.5341, 1.53, 1.7995, 2.1078, 2.1167, 2.1224, 2.1206, 2.1199]
  out "error out (frontpanel screenshots)":errorcluster
  out "error out (graph operations)":errorcluster
  out "error out (monthly folder creation)":errorcluster={"status"=TRUE, "code"=10, "source"="Create Folder in CRYO_MASTER_FULL.vi<APPEND>\nC:\\LabVIEW\\DATA\\Google\\TUCAN Experiments\\KEK_cryotests_2019-2020\\data\\screenshots\\202010"}
  out "RUN Identifier 7":string="20201002_111738_PreCooling" caption="RUN Identifier"
  out "error out (notifier)":errorcluster
  # "GLOBAL STATUS/CONTROL"
  # "Global Settings"
  # "USB6210 Analog inputs Settings"
  # "USB6218 Analog inputs Settings"
  # "USB6218 Digital Output Settings"
  # "USB6218 Analog Output Settings"
  # "LSI218 Settings"
  # "LSI336 Settings"
  # "Graph screenshots"
  # "Configuration"
  # "Activated only when *FIll state* = TRUE"
  # "Activated only when *FIll state* = TRUE"
  # "Vavle Status"
  # "OPEN"
  # "CLOSED"
  # "ADCMT6240A Control/Status"
  # "ADCMT6240A Initialization"
  # "Set Currents (mA)"
  # "KIKUSUI PWR400H CTRL via USB6218"
  # "DMM configurations"
  # "DMM measurements"
  # "CAUTION: ADCMT 7351 does not have 4-wire resistance measurement function. \n 4-Wire Resistance --> 2-Wire Resistance wih Low Power for this device"
  # "Representative temperatures"
  # "Pressures / Flows"
  # "Labels"
  # "Values"
  # "Helium Levels"
types:
  T1 = cluster{"TimeArray":timestamp[], "DataArray":dbl[]}[]
  T2 = enum32{"NI USB CONFIG", "LSI CONFIG", "MEASUREMENT", "HE AUTO FILL", "VALVE/HEATER CTRL", "DMMs", "DIAGRAM", "(Plc. hld.)"}
  T3 = cluster{"Label":string, "FileFormat":string, "Active?":bool, "Physical CH":tag, " terminal\n type":i32, "ConversionType":cluster{"Type":enum16{"Raw", "SimpleProp", "CC-10_COMBINED", "CC-10_LOG", "LeakDet_EXP", "LeakDet_Mantissa", "Baratron"}, "ConversionParameters":dbl[]}, "VoltageLimits":dbl[]}[]
  T4 = cluster{"LSIName":string, "Labels":string[], "SensorLocations":enum16{"N.C.", "T3He1-1", "T3He1-2", "T3He1-3", "T3He1-4", "T3He2-1", "T3He2-2", "T3He3", "T3He4", "T3He5", "T3He6-1", "T3He6-2", "T3He7-1", "T3He7-2", "T3He8", "T3He9", "T3He10", "T4He1", "T4He2-1", "T4He2-2", "T4He3-1", "T4He3-2", "T4He3-3", "T4He3-4", "T4He4", "T4He5", "T4He6", "T4He7", "T4He8", "T4He9", "T4He10", "T1K1", "T1K2", "T1K3-1", "T1K3-2", "T1K4", "T1K5", "T1K6", "TIP1", "TIP2", "TIP3", "TIP4", "TIP5", "TIP6", "TIP7", "TTH1", "TTH2", "TTH3", "TTH4"}[], "Active?":bool, "VISA res. name":refnum<visa-resource-name>}[]
  T5 = enum32{"USB6210", "USB6218", "Temeprature (1)", "Temperature (2)", "Temperature (3)"}
  T6 = enum16{"Intialized", "Ready", "Measuring", "Terminated"}
  T7 = enum16{"Initialized", "Ready", "Measuring", "Terminated"}
  T8 = cluster{"TimeArray":timestamp[], "Filtered X":dbl[]}[]
  T9 = cluster{"TimeArray (USB6218)":timestamp[], "DataArrayConv (USB6218)":dbl[]}[]
  T10 = cluster{"Label":string, "Active?":bool, "VISA resource name":refnum<visa-resource-name>, "Device":enum16{"Agilent34401A", "ADCMT7351", "HP3478A"}, "Measurement":enum16{"DC Volts", "DC Currents", "2-Wire Resistance", "4-Wire Resistance"}, "FileFormat":string}[]
  T11 = enum16{"N.C.", "T3He1-1", "T3He1-2", "T3He1-3", "T3He1-4", "T3He2-1", "T3He2-2", "T3He3", "T3He4", "T3He5", "T3He6-1", "T3He6-2", "T3He7-1", "T3He7-2", "T3He8", "T3He9", "T3He10", "T4He1", "T4He2-1", "T4He2-2", "T4He3-1", "T4He3-2", "T4He3-3", "T4He3-4", "T4He4", "T4He5", "T4He6", "T4He7", "T4He8", "T4He9", "T4He10", "T1K1", "T1K2", "T1K3-1", "T1K3-2", "T1K4", "T1K5", "T1K6", "TIP1", "TIP2", "TIP3", "TIP4", "TIP5", "TIP6", "TIP7", "TTH1", "TTH2", "TTH3", "TTH4"}
  T12 = cluster{"LSIName":string, "Active?":bool, "LastData":dbl[], "Labels":string[]}[]
  T13 = enum16{"N.C.", "T3He1-1", "T3He1-2", "T3He1-3", "T3He1-4", "T3He2-1", "T3He2-2", "T3He3", "T3He4", "T3He5", "T3He6-1", "T3He6-2", "T3He7-1", "T3He7-2", "T3He8", "T3He9", "T3He10", "T4He1", "T4He2-1", "T4He2-2", "T4He3-1", "T4He3-2", "T4He3-3", "T4He3-4", "T4He4", "T4He5", "T4He6", "T4He7", "T4He8", "T4He9", "T4He10", "T1K1", "T1K2", "T1K3-1", "T1K3-2", "T1K4", "T1K5", "T1K6", "TIP1", "TIP2", "TIP3", "TIP4", "TIP5", "TIP6", "TIP7", "TTH1", "TTH2", "TTH3", "TTH4"}[]
  T14 = typedef "imagedata.ctl" = cluster{"image type":i32, "image depth":i32, "image":u8[], "mask":u8[], "colors":u32[], "Rectangle":cluster{"left":i16, "top":i16, "right":i16, "bottom":i16}}
  T15 = cluster{"appended array":timestamp[], "ActualCurrentArray":dbl[]}
  T16 = cluster{"appended array":timestamp[], "SetCurrentArray":dbl[]}
  T17 = cluster{"appended array":timestamp[], "SetCurrentArray":dbl[]}[]
  T18 = cluster{"TimeArray (USB6218)":timestamp[], "DataArrayConv (USB6218)":dbl[]}
  T19 = enum16{"open", "replace", "create", "open or create", "replace or create", "replace or create with confirmation"}
  T20 = cluster{"TimeArray":timestamp[], "DataArrayConv":dbl[]}[]
  T21 = cluster{"IndexArray":i64[], "TimeArray":timestamp[], "DataArrayRaw":dbl[][], "DataArrayConv":dbl[][], "LDArray":dbl[]}